vi "15-12-13 UHR-Fleezers Control (host) - 15.2.1UCB Darwin.vi"() -> ()   [LabVIEW 2014] (continued)
  T25 = enum16{"empty", "write", "read oldest (queue)", "read newest (stack)", "read all"}
  T26 = cluster{"New Image":T2, "New Image":T2, "New Image":T2, "New Image":T2, "New Image":T2}
  T27 = typedef "XDNodeRunTimeDep.lvlib/timing_clust.ctl" = cluster{"Expected End [f-1]":u64, "Actual End [f-1]":u64, "Finished Late? [f-1]":bool, "Expected End [i-1]":u64, "Actual End [i-1]":u64, "Finished Late? [i-1]":bool, "Expected Start [i]":u64, "Actual Start [i]":u64, "Expected Start [f]":u64, "Actual Start [f]":u64, "Source Name":string, "Structure Name":string, "Period":i64, "Deadline":i64, "Offset":i64, "Start":i64, "Priority":i32, "Timeout":i32, "Mode":T28, "Wakeup Reason":T29, "Error":errorcluster, "Source Type":string, "Secondary Source Type":string, "Global End Time":u64, "Global Start Time":u64, "Frame Duration":u64, "Iteration Duration":u64, "Assigned CPU":i32, "I/O Scan Engine Mode":u32}
  T28 = typedef "XDNodeRunTimeDep.lvlib/nitl_modes.ctl" = enum32{"No Change", "Process missed periods, maintain original phase", "Discard missed periods, maintain original phase", "Process missed periods, ignore original phase", "Discard missed periods, ignore original phase"}
  T29 = typedef "XDNodeRunTimeDep.lvlib/wakeup.ctl" = enum32{"Normal", "Aborted", "Asynchronous wakeup", "Timing source error", "Timed loop error", "Timeout"}
  T30 = enum32{"Status", "Sample Stage", "Syringe Pump", "Trap Control (RF)", "APD Counting", "Fluorescence Laser Control", "Trap AI", "Video", "FPGA"}
  T31 = enum32{"Status", "Sample Stage", "Syringe Pump", "Trap Control (RF)", "APD Counting", "Fluorescence Laser Control", "Trap AI", "Video", "FPGA", "Misc. Configuration"}
  T32 = enum16{"big-endian, network order", "native, host order", "little-endian"}
  T33 = enum16{"open", "replace", "create", "open or create", "replace or create", "replace or create with confirmation"}
  T34 = cluster{"Scan Range AOD (nm) 2":dbl, "Step Size AOD (nm) 2":dbl, "Scan Speed AOD (nm/s) 2":dbl, "Number of scans (AOD) 2":u16, "Label":string}
  T35 = cluster{"[0]":dbl, "[1]":dbl, "[2]":dbl, "[3]":dbl, "[4]":dbl, "[5]":dbl}
  T36 = cluster{"Diameter (mm)":dbl, "Units":dbl, "Volume":dbl, "Rate":dbl}
  T37 = cluster{"Left":i32, "Top":i32, "Width":u32, "Height":u32}
  T38 = cluster{cluster{"Left":i32, "Top":i32, "Width":u32, "Height":u32}}[]
  T39 = enum32{"setting", "request", "request control", "info", "statistics", "system settings", "I/O sub system", "HRT control", "camera descriptions", "device specific data", "event sub system settings", "event sub system results", "image memory manager"}
  T40 = typedef "IMAQ AVI2 Refnum.ctl" = refnum<k20>
  T41 = typedef "imagedata.ctl" = cluster{"image type":i32, "image depth":i32, "image":u8[], "mask":u8[], "colors":u32[], "Rectangle":cluster{"left":i16, "top":i16, "right":i16, "bottom":i16}}
  T42 = typedef "Sound Output Task ID.ctl" = u32
  T43 = enum32{"Normal Display", "Dual Display (APD)", "FFT", "High Res Display"}
  T44 = cluster{"Origin Pixel":cluster{"X":sgl, "Y":sgl}, "Angle Relative to Horizontal (deg)":sgl, "Axis Reference":u32}
  T45 = typedef "Simple Grid Descriptor" = cluster{"X Step":sgl, "Y Step":sgl, "Unit":T46}
  T46 = typedef "Image Unit" = enum32{"Undefined", "Angström", "Micrometer", "Millimeter", "Centimeter", "Meter", "Kilometer", "Microinch", "Inch", "Feet", "Nautical miles", "Standard miles", "Steps"}
  T47 = cluster{"averaging mode":u16, "weighting mode":u16, "number of averages":u32}
  T48 = cluster{"dB On (F)":bool, "unwrap phase (F)":bool, "convert to degree (F)":bool}
  T49 = cluster{string, string, string, string, string, string, string, string}
  T50 = cluster{string, string, string, string, string, string, string, string, string, string, string, string}
  T51 = cluster{string, string, string, string, string, string, string, string, string, string, string, string, string}
  T52 = cluster{string, string, string, string, string, string, string, string, string, string, string, string, string, string}
  T53 = cluster{"BD 1 Frequency 1 (MHz)":dbl, "BD 1 Frequency 2 (MHz)":dbl}
  T54 = cluster{"f0":dbl, "df":dbl, "magnitude":dbl[]}[][]
  T55 = cluster{"Comment (data description)":string, "Channel 1 Buffer":string, "Channel 2 Buffer":string, "Channel 3 Buffer":string, "Title":string, "DNA Construct":string, "Bead diameter":dbl, "Name":string}
diagram:
  w29 = T23 2 items=["Grayscale (U8)", "Grayscale (I16)", "Grayscale (SGL)", "Complex (CSG)", "RGB (U32)", "HSL (U32)", "RGB (U64)", "Grayscale (U16)"] ("Image Type")
  # "Settings to help prevent AOM/D damage"
  # "Initialize the FPGA DAQ card itself"
  # "Reset the DAQ card."
  # "Specify the DAQ card and the FPGA code to run"
  # "Bottom 1 Harvard"
  # "Top 3 Harvard"
  # "Center Harvard"
  n1 = case "Trap X limits" shown="\"1axis\", Default" "1axis AOM vs 2 axis AOD" {
    tunnel: [T18 {"Minimum"=0.0, "Maximum"=40.0, "Increment"=0.1} ("Min Max Inc") T18 {"Minimum"=0.0, "Maximum"=40.0, "Increment"=0.1} ("Min Max Inc") T18 {"Minimum"=60.0, "Maximum"=90.0, "Increment"=1.0} ("Min Max Inc")] -> w19
    tunnel: [T18 {"Minimum"=0.0, "Maximum"=45.0, "Increment"=1.0} ("Data Entry Limits") T18 {"Minimum"=0.0, "Maximum"=45.0, "Increment"=1.0} ("Data Entry Limits") T18 {"Minimum"=0.0, "Maximum"=50.0, "Increment"=1.0} ("Data Entry Limits")] -> w17
    frame "2axisAOD" {
      w73 = u16 300 ("DIO count 1 (ticks)")
      # "Amp Limits"
      # "Freq Limits"
      n2 = disable-structure shown="Disabled" {
        frame Disabled {
          w79 = 35.0 ("BD 1 Amplitude 1 (%)")
          w80 = 30.0 ("BD 1 Frequency 1 (MHz)")
          n3 = local write "BD 1 Frequency 1 (MHz)"(w80) -> ()
          n4 = local write "BD 1 Frequency 2 (MHz)"(w80) -> ()
          n5 = local write "BD 1 Amplitude 2 (%)"(w79) -> ()
          n6 = local write "BD 1 Amplitude 1 (%)"(w79) -> ()
          n7 = local write "BD 2 Frequency 1 (MHz)"(w80) -> ()
          n8 = local write "BD 2 Amplitude 1 (%)"(w79) -> ()
          n9 = local write "BD 2 Frequency 2 (MHz)"(w80) -> ()
          n10 = local write "BD 2 Amplitude 2 (%)"(w79) -> ()
        }
        frame Enabled {
        }
      }
      n11 = local write "All FB On/Off"(FALSE ("All FB On/Off")) -> ()
      n12 = local write "BD 2 Delay (Ticks)"(u8 108 ("BD 2 Delay (Ticks)")) -> ()
      n13 = local write "Number Interlace Sets"(u8 2 ("Number Interlace Sets")) -> ()
      n14 = local write "DIO count 2 (ticks)"(w73) -> ()
      n15 = local write "DIO count 1 (ticks)"(w73) -> ()
    }
    frame "AOD3Sets" {
      w81 = u16 200 ("DIO count 1 (ticks)")
      # "Amp Limits"
      # "Freq Limits"
      n16 = disable-structure shown="Disabled" {
        frame Disabled {
          w87 = 35.0 ("BD 1 Amplitude 1 (%)")
          w88 = 30.0 ("BD 1 Frequency 1 (MHz)")
          n17 = local write "BD 1 Frequency 1 (MHz)"(w88) -> ()
          n18 = local write "BD 1 Frequency 2 (MHz)"(w88) -> ()
          n19 = local write "BD 1 Amplitude 2 (%)"(w87) -> ()
          n20 = local write "BD 1 Amplitude 1 (%)"(w87) -> ()
          n21 = local write "BD 2 Frequency 1 (MHz)"(w88) -> ()
          n22 = local write "BD 2 Amplitude 1 (%)"(w87) -> ()
          n23 = local write "BD 2 Frequency 2 (MHz)"(w88) -> ()
          n24 = local write "BD 2 Amplitude 2 (%)"(w87) -> ()
        }
        frame Enabled {
        }
      }
      n25 = local write "All FB On/Off"(FALSE ("All FB On/Off")) -> ()
      n26 = local write "BD 2 Delay (Ticks)"(u8 0 ("BD 2 Delay (Ticks)")) -> ()
      n27 = local write "Number Interlace Sets"(u8 3 ("Number Interlace Sets")) -> ()
      n28 = local write "DIO count 2 (ticks)"(w81) -> ()
      n29 = local write "DIO count 1 (ticks)"(w81) -> ()
    }
    frame "1axis", Default {
      # "Amp Lmits"
      # "Freq Limits"
    }
  }
  n30 = xnode "Open FPGA VI Reference"("resource name"=T22 "RIO0") -> ("FPGA VI Reference Out"=w23:T24, "error out"=w22:errorcluster)  [unwired: 1 in]
  n31 = xnode "Invoke Method"("FPGA VI Reference In"=w23, "error in"=w22) -> ("FPGA VI Reference Out"=w16:T24, "error out"=→"FPGA error out":errorcluster)
  n32 = flat-sequence "Safety limits on RF frequencies and amplitudes (for AOM protection)" {
    tunnel: [w93] -> w11
    tunnel: [w92] -> w13
    tunnel: [w94] -> w14
    tunnel: [w95] -> w12
    tunnel: w19 -> [w93]
    tunnel: w17 -> [w92]
    tunnel: w16 -> [w91]
    tunnel: [w91] -> w15
    frame #0 {
      w95 = T18 {"Minimum"=0.0, "Maximum"=40.0, "Increment"=0.1} ("Min Max Inc")
      w94 = T18 {"Minimum"=0.0, "Maximum"=45.0, "Increment"=1.0} ("Data Entry Limits")
      n33 = property on="BD 2 Frequency 1 (MHz)" class="DigNum (strict)"("Data Range"=w95) -> ()  [unwired: 2 in, 2 out]
      n34 = property on="BD 2 Frequency 3 (MHz)" class="DigNum (strict)"("Data Range"=w95) -> ()  [unwired: 2 in, 2 out]
      n35 = property on="BD 2 Frequency 2 (MHz)" class="DigNum (strict)"("Data Range"=w95) -> ()  [unwired: 2 in, 2 out]
      n36 = property on="BD 1 Frequency 1 (MHz)" class="DigNum (strict)"("Data Range"=w93) -> ()  [unwired: 2 in, 2 out]
      n37 = property on="BD 1 Frequency 2 (MHz)" class="DigNum (strict)"("Data Range"=w93) -> ()  [unwired: 2 in, 2 out]
      n38 = property on="BD 1 Frequency 3 (MHz)" class="DigNum (strict)"("Data Range"=w93) -> ()  [unwired: 2 in, 2 out]
      n39 = property on="BD 2 Amplitude 1 (%)" class="DigNum (strict)"("Data Range"=w94) -> ()  [unwired: 2 in, 2 out]
      n40 = property on="BD 2 Amplitude 2 (%)" class="DigNum (strict)"("Data Range"=w94) -> ()  [unwired: 2 in, 2 out]
      n41 = property on="BD 2 Amplitude 3 (%)" class="DigNum (strict)"("Data Range"=w94) -> ()  [unwired: 2 in, 2 out]
      n42 = property on="BD 1 Amplitude 3 (%)" class="DigNum (strict)"("Data Range"=w92) -> ()  [unwired: 2 in, 2 out]
      n43 = property on="BD 1 Amplitude 2 (%)" class="DigNum (strict)"("Data Range"=w92) -> ()  [unwired: 2 in, 2 out]
      n44 = property on="BD 1 Amplitude 1 (%)" class="DigNum (strict)"("Data Range"=w92) -> ()  [unwired: 2 in, 2 out]
      "X RF Frequency Limits (MHz)" <- w93
      "X RF Amplitude Limits (%)" <- w92
      "Y RF Amplitude Limits (%)" <- w94
      "Y RF Frequency Limits (MHz)" <- w95
    }
  }
  n45 = stacked-sequence "Host initialization sequence - order matters!" {
    tunnel: w15 -> [_ w98 w193 _ w263 w271 w317 w342 w372]
    tunnel: [_ _ _ _ _ _ _ _ w372] -> w4
    tunnel: [_ _ _ _ _ _ _ _ w371] -> w20
    tunnel: w14 -> [_ _ _ _ _ _ w314 _ _]
    tunnel: w13 -> [_ _ _ _ _ _ w313 _ _]
    tunnel: w12 -> [_ _ _ _ _ _ w312 _ _]
    tunnel: w11 -> [_ _ _ _ _ _ w311 _ _]
    frame #0 {
    }
    frame #1 {
      w131 = 10.0 ("y")
      w132 = 32767.0 ("y")
      w116 = 6.0  # clock mult.
      w115 = 49152000.0  # TCXO frequ.
      # "Initialize some FPGA settings"
      n46 = Build Array("DIO count 1 (ticks)", "DIO count 2 (ticks)", "DIO count 3 (ticks)") -> (w166:u16[])
      n47 = local read "AO1"() -> (w137:dbl)
      n48 = local read "AO2"() -> (w138:dbl)
      n49 = local read "Scan Increment (MHz)"() -> (w120:dbl)
      n50 = property on="AI Count (ticks)" class="DigNum (strict)"("Val(Sgnl)"="AI Count (ticks)") -> ()  [unwired: 2 in, 2 out]
      n51 = local read "Continuous MCL Scanning"() -> (w150:bool)
      n52 = local read "Fast Scan Dir"() -> (w151:bool)
      n53 = local read "Number of scans (MCL)"() -> (w149:u64)
      n54 = Multiply(x=w137, y=w132) -> (x*y=w135:dbl)
      n55 = Multiply(x=w138, y=w132) -> (x*y=w133:dbl)
      n56 = Divide(x=40000000.0, y="AI Count (ticks)") -> (x/y=w155:dbl)
      n57 = Divide(x=w135, y=w131) -> (x/y=w136:dbl)
      n58 = Divide(x=w133, y=w131) -> (x/y=w134:dbl)
      n59 = To Word Integer(number=w136) -> (16bit integer=w139:i16)
      n60 = To Word Integer(number=w134) -> (16bit integer=w140:i16)
      n61 = Not(x=w151) -> (.not. x?=w152:bool)
      n62 = local read "Cycles/step (MCL)"() -> (w148:u64)
      n63 = Multiply(x=w120, y=1000.0) -> (x*y=w113:dbl)
      n64 = local read "Scan steps (MCL)"() -> (w147:u64)
      n65 = local write "Trap Pos FIFO Timeout"(u16 0 ("Trap Pos FIFO Timeout")) -> ()
      n66 = local read "Desired Scan Incr (V)"() -> (w145:dbl)
      n67 = local write "AI rate (Hz)"(w155) -> ()
      n68 = Scale By Power Of 2(n=48, x=w113) -> (x*2^n=w112:dbl)
      n69 = Unbundle By Name(cluster{"output high":i16, "output low":i16} {"output high"=3000, "output low"=0} ("FB output range 1")) -> ("output high"=w185:i16, "output low"=w186:i16)
      n70 = Multiply(x=w115, y=w116) -> (x*y=w117:dbl)
      n71 = Divide(x=w112, y=w117) -> (x/y=w118:dbl)
      n72 = local read "Setpoints (V)"() -> (w105:cluster{"Set 1":dbl, "Set 2":dbl})
      n73 = To Quad Integer(1:w118) -> (0:w121:i64)
      n74 = Multiply(x=w145, y=32767.0) -> (x*y=w143:dbl)
      n75 = Divide(x=w155, y="FPGA Ave.") -> (x/y=w154:dbl)
      n76 = local read "Trap Intensity PID Gains"() -> (w110:T11)
      n77 = local read "Next trap write delay (ticks)"() -> (w189:u8)
      n78 = local read "XY phase ext loop method"() -> (w190:bool)
      n79 = local write "Ave. Rate (Hz)"(w154) -> ()
      n80 = Reciprocal(x=w154) -> (1/x=w153:dbl)
      n81 = local read "Number Interlace Sets"() -> (w173:u8)
      n82 = Split 1D Array(array=w166, index=w173) -> (first subarray=w164:u16[])  [unwired: 1 out]
      n83 = Add Array Elements(numeric array=w164) -> (sum=w165:u16)
      n84 = local write "Ave. Period (s)"(w153) -> ()
      n85 = local read "# Samples/channel"() -> (w128:u32)
      n86 = local read "Number of F/B Scans (AOD)"() -> (w127:u16)
      n87 = local read "Not-Interlacing Set"() -> (w174:enum32{"Set 1", "Set 2", "Set 3"})
      n88 = To Unsigned Byte Integer(number=w174) -> (unsigned 8bit integer=w168:u8)
      n89 = Index Array(array=w166, index=w168) -> (element=w167:u16)
      n90 = local read "Feedback On/Off"() -> (w102:cluster{"Set 1":bool, "Set 2":bool})
      n91 = local read "BD 2 Delay (Ticks)"() -> (w188:u8)
      n92 = local read "BD 1 Delay (ticks)"() -> (w187:u8)
      n93 = local read "Scan steps (AOD)"() -> (w122:u64)
      n94 = local read "All FB On/Off"() -> (w101:bool)
      n95 = local read "Cycles/step (AOD)"() -> (w123:u64)
      n96 = Divide(x=w143, y=10.0) -> (x/y=w144:dbl)
      n97 = Multiply(x=w122, y=w123) -> (x*y=w124:u64)
      n98 = Unbundle By Name(w110) -> ("proportional gain (Kc)"=w181:i16, "integral gain (Kc*Ts/Ti)"=w182:i16, "derivative gain (Kc*Td/Ts)"=w183:i16)
      n99 = Multiply(x=3276.7, y=w105) -> (x*y=w106:cluster{"Set 1":dbl, "Set 2":dbl})
      n100 = To Word Integer(number=w144) -> (16bit integer=w146:i16)
      n101 = Multiply(x=w124, y=u64 2) -> (x*y=w126:u64)
      n102 = To Word Integer(number=w106) -> (16bit integer=w107:cluster{"Set 1":i16, "Set 2":i16})
      n103 = Multiply(x=w126, y=w127) -> (x*y=w129:u64)
      n104 = local read "Sets to FIFO (Traps)"() -> (w177:T17)
      n105 = Divide(x=w129, y=w128) -> (x/y=w130:dbl)
      n106 = Unbundle By Name(w107) -> ("Set 1"=w108:i16, "Set 2"=w109:i16)
      n107 = local read "2D or 1D Scan"() -> (w163:bool)
      n108 = local write "Data points/scans"(w129) -> ()
      n109 = local read "Scan BD"() -> (w111:bool)
      n110 = And(x=w102, y=w101) -> (x .and. y?=w103:cluster{"Set 1":bool, "Set 2":bool})
      n111 = local write "Data points/scan (f/b)"(w126) -> ()
      n112 = local read "N Acq Sets (Traps + Fl.)"() -> (w159:i16)
      n113 = local write "N sets should be saved"(w130) -> ()
      n114 = local read "FPGA error out"() -> (w97:errorcluster)
      n115 = Unbundle By Name(w103) -> ("Set 1"=w99:bool, "Set 2"=w100:bool)
      n116 = local read "Interlace"() -> (w172:bool)
      n117 = Select(t=w165, s=w172, f=w167) -> (s? t:f=w175:u16)
      n118 = local write "Update Count (MCL)"(w175) -> ()
      n119 = local write "Total Counts (ticks)"(w175) -> ()
      n120 = Unbundle By Name(w177) -> ("Set 1"=w178:bool, "Set 2"=w179:bool, "Set 3"=w180:bool)
      n121 = property on="2D or 1D Scan" class="Bool (strict)"("Val(Sgnl)"=w163) -> ()  [unwired: 2 in, 2 out]
      n122 = xnode "Read/Write Control"("FPGA VI Reference In"=w98, "error in"=w97, "ai count"="AI Count (ticks)", "Interlace ON/OFF"=w172, "Number Interlace Cycles"=w173, "Set 1"=w178, "Set 2"=w179, "Set 3"=w180, "FB On/Off Set 1"=w99, "FB On/Off Set 2"=w100, "Interlace Off Parameters"=w174, "FB Setpoint Set 1"=w108, "FB Setpoint Set 2"=w109, "P1"=w181, "I1"=w182, "D1"=w183, "FB1 output high"=w185, "FB1 output low"=w186, "Cycles per step"=w123, "Scan BD"=w111, "Number of scans"=w127, "Scan steps"=w122, "Scan freq.  increment"=w121, "AO1"=w139, "AO2"=w140, "Scan freq.  increment (MCL)"=w146, "Scan steps (MCL)"=w147, "Cycles per step (MCL)"=w148, "Number of scans (MCL)"=w149, "MCL count"=w175, "Cont. Scan (MCL)"=w150, "MCL Scan Axis"=w152, "1D or 2D Scan?"=w163, "N of AI1 Int Acq Sets"=w159, "Amp switch delay"="Amp switch delay", "Swap F1 and F2"="Swap F1 and F2", "APD to FIFO"=FALSE, "DIO count 1 (ticks)"="DIO count 1 (ticks)", "DIO count 2 (ticks)"="DIO count 2 (ticks)", "DIO count 3 (ticks)"="DIO count 3 (ticks)", "BD 1 Delay (ticks)"=w187, "BD 2 Delay (Ticks)"=w188, "Next trap write delay (ticks)"=w189, "XY phase ext loop method"=w190) -> ("error out"=w96:errorcluster)  [unwired: 1 in, 1 out]
      n123 = local write "FPGA error out"(w96) -> ()
    }
    frame #2 {
      # "Initialize some more FPGA settings"
      n124 = local read "Laser interlacing mode"() -> (w194:enum32{"Laser ON", "Laser OFF", "Interlace"})
      n125 = local read "Green Laser ON"() -> (w195:bool)
      n126 = local read "Trap Pos. FB Range"() -> (w217:T14)
      n127 = local read "Trap Pos. FB Gains"() -> (w218:T13)
      n128 = Multiply(x="Green Intensity % (FB OFF)", y=655.35) -> (x*y=w200:dbl)
      n129 = local read "Invert laser interlacing"() -> (w237:bool)
      n130 = local read "Trap Pos. AI1 X Pre-scale"() -> (w211:u16)
      n131 = Multiply(x="Green FB Setpoint (mV)", y=3.2767) -> (x*y=w203:dbl)
      n132 = local read "Trap Pos FB Int Count"() -> (w213:u16)
      n133 = local read "Differential FB?"() -> (w216:bool)
      n134 = local read "Neg. TTrig FPGA"() -> (w214:bool)
      n135 = Multiply(x="Red FB Setpoint (mV)", y=3.2767) -> (x*y=w229:dbl)
      n136 = To Unsigned Word Integer(number=w200) -> (unsigned 16bit integer=w202:u16)
      n137 = Multiply(x="Red Intensity % (FB OFF)", y=655.35) -> (x*y=w233:dbl)
      n138 = To Word Integer(number=w203) -> (16bit integer=w205:i16)
      n139 = Unbundle By Name("Green FB Gains") -> ("proportional gain (Kc)"=w226:i16, "integral gain (Kc*Ts/Ti)"=w227:i16, "derivative gain (Kc*Td/Ts)"=w228:i16)
      n140 = Unbundle By Name("Red FB Gains") -> ("proportional gain (Kc)"=w240:i16, "integral gain (Kc*Ts/Ti)"=w241:i16, "derivative gain (Kc*Td/Ts)"=w242:i16)
      n141 = case shown="False" w195 {
        tunnel: w194 -> [_ w245]
        tunnel: [enum32{"Laser ON", "Laser OFF", "Interlace"}."Laser OFF" ("Green laser mode") w245] -> w238
        frame False {
        }
        frame True {
        }
      }
      n142 = To Word Integer(number=w229) -> (16bit integer=w232:i16)
      n143 = Unbundle By Name(w218) -> ("proportional gain (Kc)"=w222:fxp<+/-,16,8>, "integral gain (Kc*Ts/Ti)"=w223:fxp<+/-,16,8>, "derivative gain (Kc*Td/Ts)"=w224:fxp<+/-,16,8>)
      n144 = To Unsigned Word Integer(number=w233) -> (unsigned 16bit integer=w236:u16)
      n145 = Unbundle By Name(w217) -> ("output high"=w219:fxp<+/-,16,1>, "output low"=w221:fxp<+/-,16,1>)
      n146 = local read "Trap Pos FB Monitor\nT1 or T2"() -> (w206:bool)
      n147 = local read "Trap Pos FB Negate Action"() -> (w207:bool)
      n148 = local read "Trap Pos. FB Offset Factor"() -> (w208:i64)
      n149 = local read "Trap Pos. FB Mult Factor"() -> (w209:i64)
      n150 = local read "FPGA error out"() -> (w191:errorcluster)
      n151 = xnode "Read/Write Control"("FPGA VI Reference In"=w193, "error in"=w191, "Invert GI 2"=w237, "Operating Mode 2"=w238, "P3"=w226, "I3"=w227, "D3"=w228, "Green FB Setpoint"=w205, "Green FB On/Off"="Green FB On/Off", "Current Out"=w202, "Green int current ON count adj"="Green int current ON count adj", "Operating Mode"=w238, "Invert GI"=w237, "Trap Pos FB Monitor T1 or T2"=w206, "Trap Pos FB Negate Action"=w207, "Trap Pos. FB Offset Factor"=w208, "Trap Pos. FB Mult Factor"=w209, "Force feedback"=FALSE, "AI1 X Scale"=w211, "Trap Pos to FIFO"=TRUE, "Trap Pos FB Int Count"=w213, "TTrig Negate Pos"=w214, "FB Trig Integrate"="FB Trig Integrate", "Diff FB Measurement?"=w216, "Negate Diff?"="Negate Diff?", "P2"=w222, "I2"=w223, "D2"=w224, "FB2 output high"=w219, "FB2 output low"=w221, "Red FB Setpoint"=w232, "RI Current Out"=w236, "Red Laser Operating Mode"=w238, "RI Operating Mode 2"=w238, "Invert RI 2"=w237, "Invert RI"=w237, "P4"=w240, "I4"=w241, "D4"=w242, "Red FB On/Off"="Red FB On/Off") -> ("error out"=w192:errorcluster)  [unwired: 1 out]
      n152 = local write "FPGA error out"(w192) -> ()
    }
    frame #3 {
      # "Initialize more settings. Should stop using event loops to initialize."
      # "What are these?"
      n153 = stacked-sequence {
        frame #0 {
          w248 = T25."empty" ("mode")
          # "Clear external fluorescence triggering FIFO"
          # "APD loop counts"
          # "Fluorescence loop counts (rates)"
          n154 = local read "APD Integration Time (s)"() -> (w250:dbl)
          n155 = local read "Interlace ON count"() -> (w251:u16)
          n156 = call "Smart Buffer (DBL) 1.vi"("mode"=w248) -> ()  [unwired: 5 in, 6 out]
          n157 = call "Smart Buffer (DBL) 2.vi"("mode"=w248) -> ()  [unwired: 5 in, 6 out]
          n158 = property on="APD Integration Time (s)" class="DigNum (strict)"("Val(Sgnl)"=w250) -> ()  [unwired: 2 in, 2 out]
          n159 = property on="Interlace ON count" class="DigNum (strict)"("Val(Sgnl)"=w251) -> ()  [unwired: 2 in, 2 out]
          "Number of APDs" <- 3.0 ("Number of APDs")
        }
        frame #1 {
          # "Number of APDs affects\nAPD DMA transfer"
          # "General settings for all lasers:"
          # "And includes all laser\nON/OFF settings"
          # "Fluorescent lasers settings:"
          # "Blue laser settings:"
          n160 = local read "Laser interlacing mode"() -> (w253:enum32{"Laser ON", "Laser OFF", "Interlace"})
          n161 = local read "Invert laser interlacing"() -> (w252:bool)
          n162 = local read "Blue FB On/Off"() -> (w254:bool)
          n163 = property on="Blue FB On/Off" class="Bool (strict)"("Val(Sgnl)"=w254) -> ()  [unwired: 2 in, 2 out]
          n164 = property on="Invert laser interlacing" class="Bool (strict)"("Val(Sgnl)"=w252) -> ()  [unwired: 2 in, 2 out]
          n165 = property on="Laser interlacing mode" class="RadioBtnsControl (strict)"("Val(Sgnl)"=w253) -> ()  [unwired: 2 in, 2 out]
        }
        frame #2 {
          w255 = path "E:/Home/wheeler/Comstock-LabView-Link.udl" ("connection information")
          # "Initialize the database connection"
          n166 = disable-structure shown="Disabled" {
            disable-tunnel: [w258 _] -> w256
            disable-tunnel: w255 -> [w257 _]
            frame Disabled {
              n167 = call-poly <vilib>:"DB Tools Open Connection.vi"("connection information"=w257) -> ("connection reference"=w258:T19)  [unwired: 7 in, 1 out]
            }
            frame Enabled {
            }
          }
          "connection reference" <- w256
          n168 = local write "connection reference"(w256) -> ()
          n169 = local write "Database link"(w255) -> ()
        }
        frame #3 {
          # "Load active calibration to fpga"
          n170 = local read "Base N trap periods"() -> (w260:u32)
          n171 = local read "T1 Osc Enable"() -> (w259:bool)
          n172 = property on="T1 Osc Enable" class="Bool (strict)"("Val(Sgnl)"=w259) -> ()  [unwired: 2 in, 2 out]
          n173 = property on="Base N trap periods" class="DigNum (strict)"("Val(Sgnl)"=w260) -> ()  [unwired: 2 in, 2 out]
        }
      }
      n174 = local write "Offset (nm)"(0.0 ("Offset (nm)")) -> ()
      n175 = local write "Bead Mean (nm)"(0.0 ("Bead Mean (nm)")) -> ()
    }
    frame #4 {
      # "Set FIFO size and run FPGA"
      n176 = local read "FPGA error out"() -> (w262:errorcluster)
      n177 = xnode "Invoke Method"("FPGA VI Reference In"=w263, "error in"=w262, "Requested Depth"="Trap AI FIFO Depth") -> ("FPGA VI Reference Out"=w267:T24, "error out"=w268:errorcluster)  [unwired: 1 out]
      n178 = xnode "Invoke Method"("FPGA VI Reference In"=w267, "error in"=w268, "Requested Depth"="Trap Position FIFO Depth") -> ("FPGA VI Reference Out"=w265:T24, "error out"=w264:errorcluster)  [unwired: 1 out]
      n179 = xnode "Invoke Method"("FPGA VI Reference In"=w265, "error in"=w264) -> ("error out"=w261:errorcluster)  [unwired: 1 in, 1 out]
      n180 = local write "FPGA error out"(w261) -> ()
    }
    frame #5 {
      # "Adjust FPGA timing loop phases"
      n181 = flat-sequence "Initial FPGA Loop Relative Phase Adjustment" {
        tunnel: "Initial Phase Adjustment (AI1)" -> [w302]
        tunnel: "Initial Phase Adjustment (GI)" -> [w301]
        tunnel: "Initial Phase Adj. (MCL)" -> [w300]
        tunnel: [w303] -> w287
        tunnel: [w299] -> w286
        tunnel: "Initial Phase Adjustment (APD Acq)" -> [w298]
        tunnel: "Initial Phase Adjustment (APD 1 Gate)" -> [w297]
        tunnel: "Initial Phase Adjustment (Green FB)" -> [w296]
        tunnel: "Initial Phase Adjustment (GI) 2" -> [w295]
        tunnel: "Initial Phase Adjustment (APD 2 Gate)" -> [w294]
        tunnel: "Initial Phase Adjustment (RI)" -> [w293]
        tunnel: "Initial Phase Adjustment (BI DO)" -> [w292]
        tunnel: "Initial Phase Adjustment (BI AO)" -> [w291]
        tunnel: "Initial Phase Adjustment (APD 3 Gate)" -> [w290]
        tunnel: w271 -> [w289]
        tunnel: w287 -> [w305]
        tunnel: [w306] -> w285
        tunnel: w286 -> [w306]
        tunnel: [w305] -> w284
        tunnel: w285 -> [w310]
        tunnel: w284 -> [w309]
        tunnel: [w307] -> w270
        frame #0 {
          n182 = local read "FPGA error out"() -> (w288:errorcluster)
          n183 = xnode "Read/Write Control"("FPGA VI Reference In"=w289, "error in"=w288, "Phase count adjustment"=w302, "Phase count adjustment (GI)"=w301, "Phase count adjustment (MCL)"=w300, "Phase Count Adjustment (APD Acq)"=w298, "Phase count adjustment (APD 1 Gate)"=w297, "Phase count adjustment (APD 2 Gate)"=w294, "Phase count adjustment (Green FB)"=w296, "Phase count adjustment (GI) 2"=w295, "Phase count adjustment (RI)"=w293, "Phase count adjustment (BI AO)"=w291, "Phase count adjustment (BI D)"=w292, "Phase count adjustment (APD 3 Gate)"=w290) -> ("FPGA VI Reference Out"=w299:T24, "error out"=w303:errorcluster)
        }
        frame #1 {
          n184 = Wait (ms)(milliseconds to wait=u32 100) -> ()  [unwired: 1 out]
        }
        frame #2 {
          w308 = TRUE
          n185 = xnode "Read/Write Control"("FPGA VI Reference In"=w310, "error in"=w309, "+ phase"=w308, "+ phase (GI)"=w308, "+ phase (MCL)"=w308, "+ phase (APD Acq)"=w308, "+ phase (APD 1 Gate)"=w308, "+ phase (APD 2 Gate)"=w308, "+ phase (Green FB)"=w308, "+ phase (GI) 2"=w308, "+ phase (RI)"=w308, "+ phase (BI AO)"=w308, "+ phase (BI D)"=w308, "+ phase (APD 3 Gate)"=w308) -> ("error out"=w307:errorcluster)  [unwired: 1 out]
        }
      }
      n186 = local write "FPGA error out"(w270) -> ()
    }
    frame #6 {
      # "Initialize trap RF synth board and set initial frequencies and amplitudes"
      n187 = local read "FPGA error out"() -> (w316:errorcluster)
      n188 = call "Initialize RF boards - interlace 3.vi"("error in"=w316, "FPGA VI Reference In"=w317) -> ("error out"=w318:errorcluster, "FPGA VI Reference Out"=w339:T24)
      n189 = call "set RF board frequency - interlace.vi"("Board 2 Frequency Limits"=w312, "Board 1 Frequency Limits"=w311, "error in"=w318, "FPGA VI Reference In"=w339, "Board 2 Frequency 3 (MHz)"="BD 2 Frequency 3 (MHz)", "Board 1 Frequency 3 (MHz)"="BD 1 Frequency 3 (MHz)", "Board 2 Frequency 2 (MHz)"="BD 2 Frequency 2 (MHz)", "Board 2 Frequency 1 (MHz)"="BD 2 Frequency 1 (MHz)", "Board 1 Frequency 2 (MHz)"="BD 1 Frequency 2 (MHz)", "Board 1 Frequency 1  (MHz)"="BD 1 Frequency 1 (MHz)") -> ("error out"=w322:errorcluster, "FPGA VI Reference Out"=w321:T24)
      n190 = call "set RF board amplitude - interlace.vi"("Board 2 Amplitude Limits"=w314, "Board 1 Amplitude Limits"=w313, "error in"=w322, "FPGA VI Reference In"=w321, "Board 2 Amplitude 3 (%)"="BD 2 Amplitude 3 (%)", "Board 1 Amplitude 3 (%)"="BD 1 Amplitude 3 (%)", "Board 2 Amplitude 2 (%)"="BD 2 Amplitude 2 (%)", "Board 2 Amplitude 1 (%)"="BD 2 Amplitude 1 (%)", "Board 1 Amplitude 2 (%)"="BD 1 Amplitude 2 (%)", "Board 1 Amplitude 1 (%)"="BD 1 Amplitude 1 (%)") -> ("error out"=w315:errorcluster)  [unwired: 1 out]
      n191 = Subtract(x="BD 1 Frequency 1 (MHz)", y="BD 1 Frequency 2 (MHz)") -> (x-y=w329:dbl)
      n192 = Subtract(x="BD 2 Frequency 1 (MHz)", y="BD 2 Frequency 2 (MHz)") -> (x-y=w330:dbl)
      n193 = local write "FPGA error out"(w315) -> ()
      n194 = Square(x=w330) -> (x^2=w332:dbl)
      n195 = Square(x=w329) -> (x^2=w331:dbl)
      n196 = Add(x=w331, y=w332) -> (x+y=w333:dbl)
      n197 = Square Root(x=w333) -> (sqrt(x)=w334:dbl)
      n198 = local write "Trap Delta (MHz)"(w334) -> ()
    }
    frame #7 {
      n199 = local read "FPGA error out"() -> (w341:errorcluster)
      n200 = flat-sequence {
        tunnel: [w356] -> w346
        tunnel: [w355] -> w345
        tunnel: w342 -> [w348]
        tunnel: w341 -> [w347]
        tunnel: [w360] -> w344
        tunnel: w346 -> [w360]
        tunnel: [w359] -> w343
        tunnel: w345 -> [w359]
        tunnel: w344 -> [w368]
        tunnel: w343 -> [w367]
        tunnel: [w362] -> w340
        frame #0 {
          w349 = FALSE ("Retract Pump 3")
          n201 = local read "Trap 1 (ON/OFF)"() -> (w350:bool)
          n202 = xnode "Read/Write Control"("FPGA VI Reference In"=w348, "error in"=w347, "Direct RF Box  Communication"=FALSE) -> ("FPGA VI Reference Out"=w356:T24, "error out"=w355:errorcluster)
          n203 = local write "Saving..."(FALSE ("Saving Data")) -> ()
          n204 = local write "Stop All"(FALSE ("Stop All")) -> ()
          n205 = local write "Retract Pump 1"(w349) -> ()
          n206 = local write "Retract Pump 3"(w349) -> ()
          n207 = local write "Index"(1.0 ("Index")) -> ()
          n208 = property on="Trap 1 ON" class="Bool (strict)"("Value"=w350) -> ()  [unwired: 2 in, 2 out]
          "Manipulating Trap" <- FALSE ("Manipulating Trap")
        }
        frame #1 {
          n209 = local read "Trap 2 (ON/OFF)"() -> (w358:bool)
          n210 = Wait (ms)(milliseconds to wait=u32 10) -> ()  [unwired: 1 out]
          n211 = property on="Trap 2 ON" class="Bool (strict)"("Val(Sgnl)"=w358) -> ()  [unwired: 2 in, 2 out]
        }
        frame #2 {
          n212 = local read "Scan Range (nm)"() -> (w363:dbl)
          n213 = xnode "Read/Write Control"("FPGA VI Reference In"=w368, "error in"=w367, "FPGA Controls  RF Box"=TRUE ("Direct RF Box  Communication")) -> ("error out"=w362:errorcluster)  [unwired: 1 out]
          n214 = call "Update messages.vi"("Message to add"="UHR-Fleezers ready.", "Old message string"="") -> ("New message string"=w366:string)
          n215 = local write "Messages"(w366) -> ()
          n216 = property on="Scan Range (nm)" class="DigNum (strict)"("Val(Sgnl)"=w363) -> ()  [unwired: 2 in, 2 out]
        }
      }
      n217 = local write "FPGA error out"(w340) -> ()
    }
    frame #8 {
      # "Wait 5 s for all the event loops still being executed to finish."
      n218 = Wait (ms)(milliseconds to wait=u32 5000) -> ()  [unwired: 1 out]
      n219 = local read "FPGA error out"() -> (w371:errorcluster)
    }
  }
  n220 = disable-structure shown="Disabled" {
    disable-tunnel: [w404 _] -> w52
    disable-tunnel: [w401 _] -> w41
    disable-tunnel: [w400 _] -> w40
    disable-tunnel: [w395 _] -> w36
    disable-tunnel: [w394 _] -> w35
    disable-tunnel: [w393 _] -> w34
    disable-tunnel: [w392 _] -> w33
    disable-tunnel: [w389 _] -> w25
    disable-tunnel: [w384 _] -> w3
    disable-tunnel: [w377 _] -> w2
    disable-tunnel: [w374 _] -> w1
    frame Disabled {
      w376 = u16 20 items=["1.0"=10, "1.5"=15, "2.0"=20] ("stop bits (10: 1 bit)")
      w387 = u16 20 items=["1.0"=10, "1.5"=15, "2.0"=20] ("stop bits (10: 1 bit)")
      w390 = u16 10 items=["1.0"=10, "1.5"=15, "2.0"=20] ("stop bits (10: 1 bit)")
      w396 = u16 20 items=["1.0"=10, "1.5"=15, "2.0"=20] ("stop bits (10: 1 bit)")
      w398 = u16 20 items=["1.0"=10, "1.5"=15, "2.0"=20] ("stop bits (10: 1 bit)")
      w402 = u16 20 items=["1.0"=10, "1.5"=15, "2.0"=20] ("stop bits (10: 1 bit)")
      # "Bottom 1 Harvard"
      # "Top 3 Harvard"
      # "Center Harvard"
      n221 = call-poly "VISA Configure Serial Port"("VISA resource name"=refnum<visa-resource-name> "COM2", "baud rate (9600)"=u32 9600, "stop bits (10: 1 bit)"=w387) -> ("VISA resource name out"=w377:refnum<visa-resource-name>, "error out"=→"Preamp Error Out":errorcluster)  [unwired: 4 in, 7 out]
      n222 = call-poly "VISA Configure Serial Port"("VISA resource name"=refnum<visa-resource-name> "COM2", "baud rate (9600)"=u32 9600, "stop bits (10: 1 bit)"=w376) -> ("VISA resource name out"=w374:refnum<visa-resource-name>)  [unwired: 4 in, 8 out]
      n223 = call-poly "VISA Configure Serial Port"("VISA resource name"=refnum<visa-resource-name> "COM7", "baud rate (9600)"=u32 115200, "stop bits (10: 1 bit)"=w390) -> ("VISA resource name out"=w389:refnum<visa-resource-name>, "error out"=w388:errorcluster)  [unwired: 4 in, 7 out]
      n224 = call-poly "VISA Configure Serial Port"("VISA resource name"=refnum<visa-resource-name> "COM5", "baud rate (9600)"=u32 115200, "stop bits (10: 1 bit)"=w396) -> ("VISA resource name out"=w393:refnum<visa-resource-name>, "error out"=w392:errorcluster)  [unwired: 4 in, 7 out]
      n225 = call-poly "VISA Configure Serial Port"("VISA resource name"=refnum<visa-resource-name> "COM4", "baud rate (9600)"=u32 115200, "stop bits (10: 1 bit)"=w398) -> ("VISA resource name out"=w395:refnum<visa-resource-name>, "error out"=w394:errorcluster)  [unwired: 4 in, 7 out]
      n226 = call-poly "VISA Configure Serial Port"("VISA resource name"=refnum<visa-resource-name> "COM6", "baud rate (9600)"=u32 115200, "stop bits (10: 1 bit)"=w402) -> ("VISA resource name out"=w400:refnum<visa-resource-name>, "error out"=w401:errorcluster)  [unwired: 4 in, 7 out]
      n227 = call-poly "VISA Configure Serial Port"("VISA resource name"=refnum<visa-resource-name> "COM1") -> ("VISA resource name out"=w384:refnum<visa-resource-name>, "error out"=w404:errorcluster)  [unwired: 5 in, 8 out]
      "Stage Control Serial Error" <- w404
      n228 = local write "Blue Error Out"(w388) -> ()
    }
    frame Enabled {
    }
  }
  n229 = call "IMAQ Create"("Image Name"="APD 1 Image", "Image Type"=w29) -> ("New Image"=w46:T2)  [unwired: 3 in, 1 out]
  n230 = call "IMAQ Create"("Image Name"="APD 2 Image", "Image Type"=w29) -> ("New Image"=w45:T2)  [unwired: 3 in, 1 out]
  n231 = call "IMAQ Create"("Image Name"="APD 3 Image", "Image Type"=w29) -> ("New Image"=w28:T2)  [unwired: 3 in, 1 out]
  n232 = call "IMAQ Create"("Image Name"="Det. X Image", "Image Type"=w29) -> ("New Image"=w44:T2)  [unwired: 3 in, 1 out]
  n233 = call "IMAQ Create"("Image Name"="Det. Y Image", "Image Type"=w29) -> ("New Image"=w43:T2)  [unwired: 3 in, 1 out]
  n234 = Bundle("New Image"=w46, "New Image"=w45, "New Image"=w28, "New Image"=w44, "New Image"=w43) -> (w42:T26)  [unwired: 1 in]
  n235 = node-c288() -> (w49:T27)  [unwired: 4 in]
  n236 = timed-loop "Run Scripts, including: stage motion" {
    tunnel: w52 -> [w415]
    tunnel: w3 -> [w416]
    tunnel: [w416] -> w51
    tunnel: [w415] -> w50
    timing: w49 -> [_]
    timing-out: [_] -> w48
    tunnel: w40 -> [w414]
    tunnel: w41 -> [w413]
    tunnel: w36 -> [w410]
    tunnel: w35 -> [w409]
    tunnel: w34 -> [w411]
    tunnel: w33 -> [w412]
    tunnel: w25 -> [w408]
    tunnel: w15 -> [w407]
    tunnel: w2 -> [w406]
    tunnel: w1 -> [w405]
    stop <- w417 stop-if-true
    n237 = node-c288() -> ()  [unwired: 1 in, 1 out]
    n238 = event shown="[0] \"Set Position\", \"Set Position 2\", \"Set Position 3\", \"Set Position 4\", \"Set Position 5\", \"Set Position 1\", \"Set Position 6\": Value Change" {
      selector: _ -> [_ _ _ _ _ _ _ _ _ _ _ _ _ _ _ _ _ _ _ _ _ _ _ _ _ _ _]
      dyn-events: _ -> [_ _ _ _ _ _ _ _ _ _ _ _ _ _ _ _ _ _ _ _ _ _ _ _ _ _ _]
      timeout: _ -> [_ _ _ _ _ _ _ _ _ _ _ _ _ _ _ _ _ _ _ _ _ _ _ _ _ _ _]
      tunnel: ["Set Position" "Move to Position" _ _ _ _ _ _ "Read Harvard" _ _ _ _ _ _ _ _ "Got ADig bead" "Force FB Data\nScript" _ "Got DNA bead" "Take Stepping Data" _ "Take Detection Laser\nImage" _ _ _] -> _
      tunnel: [_ _ _ _ _ _ _ _ _ _ _ _ _ _ _ _ _ _ _ _ _ _ _ _ _ w1319 _] -> w417
      tunnel: w415 -> [w436 w444 w457 w487 _ _ _ _ _ w624 w658 w684 w716 w800 w829 w961 w988 _ w1024 _ _ _ _ _ _ _ _]
      tunnel: w416 -> [w437 w445 w458 w488 _ _ _ _ _ w625 w659 w685 w717 w801 w830 w962 w989 _ w1025 _ _ _ _ _ _ _ _]
      tunnel: w414 -> [_ _ _ _ _ _ _ _ w609 _ _ _ _ _ _ _ _ _ _ _ _ _ _ _ _ _ _]
      tunnel: w413 -> [_ _ _ _ _ _ _ _ w608 _ _ _ _ _ _ _ _ _ _ _ _ _ _ _ _ _ _]
      tunnel: w412 -> [_ _ _ _ _ _ _ _ _ _ _ _ _ _ _ _ _ _ _ _ _ _ _ _ _ _ _]
      tunnel: w411 -> [_ _ _ _ _ _ _ _ _ _ _ _ _ _ _ _ _ _ _ _ _ _ _ _ _ _ _]
      tunnel: w410 -> [_ _ _ _ _ _ _ _ _ _ _ _ _ _ _ _ _ _ _ _ _ _ _ _ _ _ _]
      tunnel: w409 -> [_ _ _ _ _ _ _ _ _ _ _ _ _ _ _ _ _ _ _ _ _ _ _ _ _ _ _]
      tunnel: w408 -> [_ _ _ _ w515 w522 w550 w569 _ _ _ _ _ _ _ _ _ _ _ _ _ _ _ _ _ w1318 _]
      tunnel: w407 -> [_ _ _ _ _ _ _ _ _ _ _ _ _ _ _ _ _ _ _ _ _ _ _ _ w1185 _ _]
      tunnel: w406 -> [_ _ _ _ _ _ _ _ _ _ _ _ _ _ _ _ _ _ _ _ _ _ _ _ _ _ w1329]
      tunnel: w405 -> [_ _ _ _ _ _ _ _ _ _ _ _ _ _ _ _ _ _ _ _ _ _ _ _ _ _ w1324]
      event "Set Position", "Set Position 2", "Set Position 3", "Set Position 4", "Set Position 5", "Set Position 1", "Set Position 6": Value Change {
        n239 = event-data() -> ()  [unwired: 1 in, 5 out]
        n240 = Build Array("Set Position 1", "Set Position 2", "Set Position 3", "Set Position 4", "Set Position 5", "Set Position 6") -> (w435:bool[])
        n241 = Boolean Array To Number(Boolean array=w435) -> (number=w434:u32)
        n242 = Logarithm Base 2(1:w434) -> (0:w426:dbl)
        n243 = call "Read Stage Position.vi"("error in"=w436, "VISA resource name in"=w437) -> ("Current Position"=w441:cluster{dbl, dbl, dbl}, "error out"=w440:errorcluster)  [unwired: 2 out]
        n244 = Decrement(x="Position") -> (x-1=w424:dbl)
        n245 = Greater Or Equal?(x=w426, y=0.0) -> (x >= y?=w427:bool)
        n246 = Cluster To Array(cluster=w441) -> (array=w438:dbl[])
        n247 = local write "Stage Control Serial Error"(w440) -> ()
        n248 = Select(t=w426, s=w427, f=w424) -> (s? t:f=w423:dbl)
        n249 = Increment(x=w423) -> (x+1=w422:dbl)
        n250 = Build Array (concatenate)(w422, w438) -> (w421:dbl[])
        n251 = Replace Array Subset(array="Saved Stage Positions", new element=w421, index (row)=w423) -> (w439:dbl[][])  [unwired: 1 in]
        n252 = local write "Saved Stage Positions"(w439) -> ()
      }
      event "Move to Position": Value Change {
        n253 = event-data() -> ()  [unwired: 1 in, 5 out]
        n254 = flat-sequence {
          tunnel: w445 -> [w449]
          tunnel: w444 -> [w448]
          frame #0 {
            n255 = local read "Saved Stage Positions"() -> (w451:dbl[][])
            n256 = local read "Position"() -> (w450:dbl)
            n257 = local write "Stage Moving"(TRUE ("Stage Moving")) -> ()
            n258 = call "move to saved stage position.vi"("error in"=w448, "Stage VISA resource name in"=w449, "Position"=w450, "Saved Stage Positions"=w451) -> ("error out"=w447:errorcluster)  [unwired: 1 out]
            n259 = local write "Stage Control Serial Error"(w447) -> ()
          }
          frame #1 {
            n260 = call <vilib>:"Beep.vi"() -> ()  [unwired: 3 in, 9 out]
            n261 = local write "Stage Moving"(FALSE ("Stage Moving")) -> ()
          }
        }
      }
      event "Move Cap. 1 (DNA Bottom)": Value Change {
        n262 = event-data() -> ()  [unwired: 1 in, 5 out]
        n263 = local write "Move Cap. 1 (DNA Bottom)"(FALSE ("Move Cap. 1 (DNA Right)")) -> ()
        n264 = flat-sequence {
          tunnel: w457 -> [w460]
          tunnel: w458 -> [w461]
          tunnel: [w461] -> w455
          tunnel: [w460] -> w454
          tunnel: w455 -> [w463]
          tunnel: w454 -> [w462]
          frame #0 {
            n265 = property on="Sample Channel\nFlow" class="Bool (strict)"("Val(Sgnl)"="Cap 1 Samp Flow ON") -> ()  [unwired: 2 in, 2 out]
          }
          frame #1 {
            n266 = local read "Saved Stage Positions"() -> (w473:dbl[][])
            n267 = local write "Stage Moving"(TRUE ("Stage Moving")) -> ()
            n268 = Array Subset(array=w473, index (row)=0 ("index"), length (row)=1 ("length"), index (col)=1 ("index"), length (col)=3 ("length")) -> (w470:dbl[][])
            n269 = Reshape Array(w470, 3 ("dimension size")) -> (w468:dbl[])
            n270 = Array To Cluster(array=w468) -> (cluster=w467:cluster{"[0]":dbl, "[1]":dbl, "[2]":dbl})
            n271 = call "Set Stage Position.vi"("Position"=w467, "error in"=w462, "VISA resource name in"=w463) -> ("error out"=w466:errorcluster)  [unwired: 2 out]
            n272 = local write "Stage Control Serial Error"(w466) -> ()
          }
          frame #2 {
            n273 = local write "Stage Moving"(FALSE ("Stage Moving")) -> ()
            n274 = case shown="True" "Cap 1 Flow ON" {
              frame False {
              }
              frame True {
                n275 = property on="Inject Pump 1" class="Bool (strict)"("Val(Sgnl)"=TRUE ("Value (Signaling)")) -> ()  [unwired: 2 in, 2 out]
              }
            }
            n276 = call <vilib>:"Beep.vi"() -> ()  [unwired: 3 in, 9 out]
          }
          frame #3 {
            n277 = property on="Sample Channel\nFlow" class="Bool (strict)"("Val(Sgnl)"=FALSE ("Value (Signaling)")) -> ()  [unwired: 2 in, 2 out]
            n278 = local read "Cap. 2 BD T1?\n(ADig T1, DNA T2)"() -> (w480:bool)
            n279 = case shown="True" w480 {
              tunnel: "Cap 1 T ON" -> [w482 w483]
              frame False {
                n280 = property on="Trap 1 (ON/OFF)" class="Bool (strict)"("Val(Sgnl)"=w482) -> ()  [unwired: 2 in, 2 out]
              }
              frame True {
                n281 = property on="Trap 2 (ON/OFF)" class="Bool (strict)"("Val(Sgnl)"=w483) -> ()  [unwired: 2 in, 2 out]
              }
            }
            n282 = property on="Got DNA bead" class="Bool"("Key Focus"=TRUE) -> ()  [unwired: 2 in, 2 out]
          }
        }
      }
      event "Move Cap. 2 (ADig Top)": Value Change {
        n283 = event-data() -> ()  [unwired: 1 in, 5 out]
        n284 = local write "Move Cap. 2 (ADig Top)"(FALSE ("Move Cap. 2 (ADig Left)")) -> ()
        n285 = flat-sequence {
          tunnel: w487 -> [w490]
          tunnel: w488 -> [w491]
          tunnel: [w491] -> w485
          tunnel: [w490] -> w484
          tunnel: w485 -> [w494]
          tunnel: w484 -> [w493]
          frame #0 {
            n286 = property on="Sample Channel\nFlow" class="Bool (strict)"("Val(Sgnl)"="Cap 2 Samp Flow ON") -> ()  [unwired: 2 in, 2 out]
          }
          frame #1 {
            w492 = FALSE ("Value (Signaling)")
            n287 = local read "Saved Stage Positions"() -> (w504:dbl[][])
            n288 = local write "Stage Moving"(TRUE ("Stage Moving")) -> ()
            n289 = Array Subset(array=w504, index (row)=1 ("index"), length (row)=1 ("length"), index (col)=1 ("index"), length (col)=3 ("length")) -> (w501:dbl[][])
            n290 = Reshape Array(w501, 3 ("dimension size")) -> (w499:dbl[])
            n291 = property on="Trap 1 (ON/OFF)" class="Bool (strict)"("Val(Sgnl)"=w492) -> ()  [unwired: 2 in, 2 out]
            n292 = property on="Trap 1 (ON/OFF)" class="Bool (strict)"("Val(Sgnl)"=w492) -> ()  [unwired: 2 in, 2 out]
            n293 = Array To Cluster(array=w499) -> (cluster=w498:cluster{"[0]":dbl, "[1]":dbl, "[2]":dbl})
            n294 = call "Set Stage Position.vi"("Position"=w498, "error in"=w493, "VISA resource name in"=w494) -> ("error out"=w497:errorcluster)  [unwired: 2 out]
            n295 = local write "Stage Control Serial Error"(w497) -> ()
          }
          frame #2 {
            n296 = local write "Stage Moving"(FALSE ("Stage Moving")) -> ()
            n297 = call <vilib>:"Beep.vi"() -> ()  [unwired: 3 in, 9 out]
            n298 = case shown="True" "Cap 2 Flow ON" {
              frame False {
              }
              frame True {
                n299 = property on="Inject Pump 3" class="Bool (strict)"("Val(Sgnl)"=TRUE ("Value (Signaling)")) -> ()  [unwired: 2 in, 2 out]
              }
            }
          }
          frame #3 {
            n300 = property on="Sample Channel\nFlow" class="Bool (strict)"("Val(Sgnl)"=FALSE ("Value (Signaling)")) -> ()  [unwired: 2 in, 2 out]
            n301 = case shown="False" "Cap. 2 BD T1?\n(ADig T1, DNA T2)" {
              tunnel: "Cap 2 T ON" -> [w513 w514]
              frame False {
                n302 = property on="Trap 2 (ON/OFF)" class="Bool (strict)"("Val(Sgnl)"=w513) -> ()  [unwired: 2 in, 2 out]
              }
              frame True {
                n303 = property on="Trap 1 (ON/OFF)" class="Bool (strict)"("Val(Sgnl)"=w514) -> ()  [unwired: 2 in, 2 out]
              }
            }
            n304 = property on="Got ADig bead" class="Bool"("Key Focus"=TRUE) -> ()  [unwired: 2 in, 2 out]
          }
        }
      }
      event "Send string\nto Blue Laser": Value Change {
        n305 = event-data() -> ()  [unwired: 1 in, 5 out]
        n306 = flat-sequence {
          tunnel: w515 -> [w516]
          frame #0 {
            n307 = call "serial write macro.vi"("String"="command string", "Delay (ms)"="Delay (ms)", "VISA resource name"=w516) -> ("read buffer"=→"read blue buffer":string, "error out"=→"Blue Error Out":errorcluster)  [unwired: 1 out]
            "command string sent" <- "command string"
          }
          frame #1 {
            n308 = local write "Send string\nto Blue Laser"(FALSE ("Send string")) -> ()
          }
        }
      }
      event "Get Blue Laser State": Value Change {
        n309 = event-data() -> ()  [unwired: 1 in, 5 out]
        n310 = local read "Delay (ms)"() -> (w523:i32)
        n311 = flat-sequence {
          tunnel: w523 -> [w531]
          tunnel: w522 -> [w534]
          tunnel: [w532] -> w527
          tunnel: [w531] -> w526
          tunnel: [w541] -> w525
          tunnel: [w538] -> w524
          tunnel: w527 -> [w539]
          tunnel: w526 -> [w538]
          tunnel: w525 -> [w547]
          tunnel: w524 -> [w545]
          frame #0 {
            w529 = "l?"
            n312 = local write "command string sent"(w529) -> ()
            n313 = call "serial write macro.vi"("String"=w529, "Delay (ms)"=w531, "VISA resource name"=w534) -> ("read buffer"=w530:string, "VISA resource name out"=w532:refnum<visa-resource-name>)  [unwired: 1 out]
            n314 = Decimal String To Number(string=w530) -> (number=w533:i32)  [unwired: 2 in, 1 out]
            n315 = Not Equal To 0?(x=w533) -> (x != 0?=→"Laser On":bool)
            n316 = local write "read blue buffer"(w530) -> ()
          }
          frame #1 {
            w536 = "games?" ("String")
            n317 = local write "command string sent"(w536) -> ()
            n318 = call "serial write macro.vi"("String"=w536, "Delay (ms)"=w538, "VISA resource name"=w539) -> ("read buffer"=w537:string, "VISA resource name out"=w541:refnum<visa-resource-name>)  [unwired: 1 out]
            n319 = Decimal String To Number(string=w537) -> (number=w540:i32)  [unwired: 2 in, 1 out]
            n320 = local write "read blue buffer"(w537) -> ()
            n321 = Not Equal To 0?(x=w540) -> (x != 0?=→"Analog Modulation":bool)
          }
          frame #2 {
            w543 = "gdmes?" ("String")
            n322 = local write "command string sent"(w543) -> ()
            n323 = call "serial write macro.vi"("String"=w543, "Delay (ms)"=w545, "VISA resource name"=w547) -> ("read buffer"=w544:string)  [unwired: 2 out]
            n324 = Decimal String To Number(string=w544) -> (number=w546:i32)  [unwired: 2 in, 1 out]
            n325 = Not Equal To 0?(x=w546) -> (x != 0?=→"Digital Modulation":bool)
            n326 = local write "read blue buffer"(w544) -> ()
          }
          frame #3 {
            n327 = local write "Get Blue Laser State"(FALSE) -> ()
          }
        }
      }
      event "Blue Laser Power (mW)\n(Constant Power Mode)", "Blue Laser Modulation\nPower (mW)": Value Change {
        n328 = event-data() -> ()  [unwired: 1 in, 5 out]
        n329 = flat-sequence {
          tunnel: w550 -> [w556]
          tunnel: [w554] -> w549
          tunnel: w549 -> [w563]
          frame #0 {
            n330 = local read "Delay (ms)"() -> (w555:i32)
            n331 = Concatenate Strings("slmp " ("string"), "Blue Laser Modulation\nPower (mW)") -> (w551:string)
            n332 = call "serial write macro.vi"("String"=w551, "Delay (ms)"=w555, "VISA resource name"=w556) -> ("read buffer"=w552:string, "error out"=w553:errorcluster, "VISA resource name out"=w554:refnum<visa-resource-name>)
            n333 = local write "command string sent"(w551) -> ()
            n334 = local write "read blue buffer"(w552) -> ()
            n335 = local write "Blue Error Out"(w553) -> ()
          }
          frame #1 {
            n336 = local read "Delay (ms)"() -> (w562:i32)
            n337 = Concatenate Strings("p " ("string"), "Blue Laser Power (mW)\n(Constant Power Mode)") -> (w559:string)
            n338 = call "serial write macro.vi"("String"=w559, "Delay (ms)"=w562, "VISA resource name"=w563) -> ("read buffer"=w560:string, "error out"=w561:errorcluster)  [unwired: 1 out]
            n339 = local write "command string sent"(w559) -> ()
            n340 = local write "read blue buffer"(w560) -> ()
            n341 = local write "Blue Error Out"(w561) -> ()
          }
        }
      }
      event "Laser interlacing mode", "Blue Laser Modulation Mode", "Blue Laser ON": Value Change {
        n342 = event-data() -> ()  [unwired: 1 in, 5 out]
        n343 = flat-sequence {
          tunnel: w569 -> [w574]
          tunnel: [w573] -> w566
          tunnel: [w579] -> w568
          tunnel: w566 -> [w582]
          tunnel: w568 -> [w594]
          tunnel: [w588] -> w567
          tunnel: w567 -> [w601]
          frame #0 {
            n344 = local read "Blue Laser ON"() -> (w571:bool)
            n345 = local read "Delay (ms)"() -> (w572:i32)
            n346 = case shown="False" w571 {
              tunnel: ["l0" "l1"] -> w570
              frame False {
              }
              frame True {
              }
            }
            n347 = call "serial write macro.vi"("String"=w570, "Delay (ms)"=w572, "VISA resource name"=w574) -> ("error out"=w575:errorcluster, "VISA resource name out"=w573:refnum<visa-resource-name>)  [unwired: 1 out]
            n348 = local write "Blue Error Out"(w575) -> ()
          }
          frame #1 {
            n349 = local read "Laser interlacing mode"() -> (w584:enum32{"Laser ON", "Laser OFF", "Interlace"})
            n350 = case shown="\"Laser ON\"" w584 {
              tunnel: ["cp" "em" "l0"] -> w578
              frame "Laser ON" {
              }
              frame "Interlace" {
              }
              frame "Laser OFF", Default {
              }
            }
            n351 = local read "Delay (ms)"() -> (w583:i32)
            n352 = call "serial write macro.vi"("String"=w578, "Delay (ms)"=w583, "VISA resource name"=w582) -> ("read buffer"=w580:string, "error out"=w581:errorcluster, "VISA resource name out"=w579:refnum<visa-resource-name>)
            n353 = local write "command string sent"(w578) -> ()
            n354 = local write "read blue buffer"(w580) -> ()
            n355 = local write "Blue Error Out"(w581) -> ()
          }
          frame #2 {
            n356 = case shown="\"Analog Modulation\"" "Blue Laser Modulation Mode" {
              tunnel: ["sdmes 0" "sdmes 1" "sdmes 1"] -> w589
              frame "Analog Modulation" {
              }
              frame "Digital + Analog Modulation" {
              }
              frame "Digital Modulation", Default {
              }
            }
            n357 = local read "Delay (ms)"() -> (w592:i32)
            n358 = call "serial write macro.vi"("String"=w589, "Delay (ms)"=w592, "VISA resource name"=w594) -> ("read buffer"=w590:string, "error out"=w591:errorcluster, "VISA resource name out"=w588:refnum<visa-resource-name>)
            n359 = local write "command string sent"(w589) -> ()
            n360 = local write "read blue buffer"(w590) -> ()
            n361 = local write "Blue Error Out"(w591) -> ()
          }
          frame #3 {
            n362 = local read "Blue Laser Modulation Mode"() -> (w603:string)
            n363 = case shown="\"Digital Modulation\", Default" w603 {
              tunnel: ["sames 1" "sames 1" "sames 0"] -> w599
              frame "Analog Modulation" {
              }
              frame "Digital + Analog Modulation" {
              }
              frame "Digital Modulation", Default {
              }
            }
            n364 = local read "Delay (ms)"() -> (w602:i32)
            n365 = local write "command string sent"(w599) -> ()
            n366 = call "serial write macro.vi"("String"=w599, "Delay (ms)"=w602, "VISA resource name"=w601) -> ("read buffer"=w600:string, "error out"=w598:errorcluster)  [unwired: 1 out]
            n367 = local write "read blue buffer"(w600) -> ()
            n368 = local write "Blue Error Out"(w598) -> ()
          }
        }
      }
      event "Read Harvard": Value Change {
        n369 = event-data() -> ()  [unwired: 1 in, 5 out]
        n370 = Concatenate Strings("write buffer", "\r") -> (w611:string)
        n371 = VISA Write(VISA resource name=w609, write buffer=w611, error in (no error)=w608) -> (VISA resource name out=w620:refnum<visa-resource-name>, error out=w619:errorcluster)  [unwired: 1 out]